vi "Dresden R2R Sputter 03.02.2018 IY24.vi"() -> ()   [LabVIEW 2009] (continued)
                                frame #1 {
                                n17950 = local read "Semi"() -> (w26326:bool)
                                n17951 = case shown="False" w26326 {
                                frame #0 {
                                n17952 = local write "Ch2_PA19"(TRUE ("PA3")) -> ()
                                n17953 = Wait Until Next ms Multiple(millisecond multiple=u32 1000) -> ()  [unwired: 1 out]
                                }
                                frame #1 {
                                }
                                }
                                }
                                }
                              }
                              frame #1 {
                              }
                            }
                          }
                          frame #14 {
                            # "CLOSE CH1-VBV"
                            n17954 = local read "Semi"() -> (w26329:bool)
                            n17955 = case shown="False" w26329 {
                              frame #0 {
                                n17956 = stacked-sequence {
                                frame #0 {
                                n17957 = local read "Semi"() -> (w26330:bool)
                                n17958 = case shown="False" w26330 {
                                frame #0 {
                                n17959 = while {
                                i -> [w26337]
                                stop <- w26331 stop-if-true
                                n17960 = Greater?(x=w26337, y=50) -> (0:w26335:bool)
                                n17961 = case shown="True" w26335 {
                                frame #0 {
                                }
                                frame #1 {
                                n17962 = local write "Semi"(TRUE ("Semi")) -> ()
                                n17963 = local write "Error Message"("Start up process  cancelled\nbecause  CH2-VBV not closed.\nPlease check  CH2-VBV connections." ("Error Message")) -> ()
                                }
                                }
                                n17964 = local read "Ch2_Ch_vbv_di"() -> (w26334:bool)
                                n17965 = case shown="True" w26334 {
                                tunnel: [TRUE FALSE] -> w26333
                                frame #0 {
                                }
                                frame #1 {
                                n17966 = Wait Until Next ms Multiple(millisecond multiple=u32 200) -> ()  [unwired: 1 out]
                                n17967 = local write "Ch2_Ch_vbv_do"(FALSE ("Ch1_Tp_bv_do")) -> ()
                                }
                                }
                                n17968 = local read "Semi"() -> (w26332:bool)
                                n17969 = Or(x=w26333, y=w26332) -> (x .or. y?=w26331:bool)
                                }
                                }
                                frame #1 {
                                }
                                }
                                }
                                frame #1 {
                                n17970 = local read "Semi"() -> (w26344:bool)
                                n17971 = case shown="False" w26344 {
                                frame #0 {
                                n17972 = local write "Ch2_PA20"(TRUE ("PA3")) -> ()
                                n17973 = Wait Until Next ms Multiple(millisecond multiple=u32 1000) -> ()  [unwired: 1 out]
                                }
                                frame #1 {
                                }
                                }
                                }
                                }
                              }
                              frame #1 {
                              }
                            }
                          }
                          frame #15 {
                            # "Close PL-VBV"
                            n17974 = local read "Semi"() -> (w26347:bool)
                            n17975 = case shown="False" w26347 {
                              frame #0 {
                                n17976 = stacked-sequence {
                                frame #0 {
                                n17977 = local read "Semi"() -> (w26348:bool)
                                n17978 = case shown="False" w26348 {
                                frame #0 {
                                n17979 = while {
                                i -> [w26355]
                                stop <- w26349 stop-if-true
                                n17980 = Greater?(x=w26355, y=50) -> (0:w26353:bool)
                                n17981 = case shown="True" w26353 {
                                frame #0 {
                                }
                                frame #1 {
                                n17982 = local write "Semi"(TRUE ("Semi")) -> ()
                                n17983 = local write "Error Message"("Start up process  cancelled\nbecause  PL-VBV not closed.\nPlease check PL2-VBV connections." ("Error Message")) -> ()
                                }
                                }
                                n17984 = local read "Ch2_Pl_vbv_di"() -> (w26352:bool)
                                n17985 = case shown="True" w26352 {
                                tunnel: [TRUE FALSE] -> w26351
                                frame #0 {
                                }
                                frame #1 {
                                n17986 = Wait Until Next ms Multiple(millisecond multiple=u32 200) -> ()  [unwired: 1 out]
                                n17987 = local write "Ch2_Pl_vbv_do"(FALSE ("Ch1_Tp_bv_do")) -> ()
                                }
                                }
                                n17988 = local read "Semi"() -> (w26350:bool)
                                n17989 = Or(x=w26351, y=w26350) -> (x .or. y?=w26349:bool)
                                }
                                }
                                frame #1 {
                                }
                                }
                                }
                                frame #1 {
                                n17990 = local read "Semi"() -> (w26362:bool)
                                n17991 = case shown="False" w26362 {
                                frame #0 {
                                n17992 = local write "Ch2_PA21"(TRUE ("PA3")) -> ()
                                n17993 = Wait Until Next ms Multiple(millisecond multiple=u32 1000) -> ()  [unwired: 1 out]
                                }
                                frame #1 {
                                }
                                }
                                }
                                }
                              }
                              frame #1 {
                              }
                            }
                          }
                          frame #16 {
                            # "OPEN TP-BV"
                            n17994 = local read "Semi"() -> (w26365:bool)
                            n17995 = case shown="False" w26365 {
                              frame #0 {
                                n17996 = stacked-sequence {
                                frame #0 {
                                n17997 = local read "Semi"() -> (w26366:bool)
                                n17998 = case shown="False" w26366 {
                                frame #0 {
                                n17999 = while {
                                i -> [w26373]
                                stop <- w26368 stop-if-true
                                n18000 = Greater?(x=w26373, y=50) -> (0:w26371:bool)
                                n18001 = case shown="True" w26371 {
                                frame #0 {
                                }
                                frame #1 {
                                n18002 = local write "Semi"(TRUE ("Semi")) -> ()
                                n18003 = local write "Error Message"("Start up process  cancelled\nbecause  TP-BV not opened.\nPlease check TP-BV2 connections." ("Error Message")) -> ()
                                }
                                }
                                n18004 = local read "Ch2_Tp_bv_di"() -> (w26367:bool)
                                n18005 = case shown="False" w26367 {
                                tunnel: [FALSE TRUE] -> w26370
                                frame #0 {
                                n18006 = Wait Until Next ms Multiple(millisecond multiple=u32 200) -> ()  [unwired: 1 out]
                                n18007 = local write "Ch2_Tp_bv_do"(TRUE ("Ch1_Tp_bv_do")) -> ()
                                }
                                frame #1 {
                                }
                                }
                                n18008 = local read "Semi"() -> (w26369:bool)
                                n18009 = Or(x=w26370, y=w26369) -> (x .or. y?=w26368:bool)
                                }
                                }
                                frame #1 {
                                }
                                }
                                }
                                frame #1 {
                                n18010 = local read "Semi"() -> (w26380:bool)
                                n18011 = case shown="False" w26380 {
                                frame #0 {
                                n18012 = local write "Ch2_PA22"(TRUE ("PA3")) -> ()
                                n18013 = Wait Until Next ms Multiple(millisecond multiple=u32 1000) -> ()  [unwired: 1 out]
                                }
                                frame #1 {
                                }
                                }
                                }
                                }
                              }
                              frame #1 {
                              }
                            }
                          }
                          frame #17 {
                            # "CLOSE CH-ATM"
                            n18014 = local read "Semi"() -> (w26383:bool)
                            n18015 = case shown="False" w26383 {
                              frame #0 {
                                n18016 = stacked-sequence {
                                frame #0 {
                                n18017 = local read "Semi"() -> (w26384:bool)
                                n18018 = case shown="False" w26384 {
                                frame #0 {
                                n18019 = while {
                                i -> [w26391]
                                stop <- w26385 stop-if-true
                                n18020 = Greater?(x=w26391, y=50) -> (0:w26389:bool)
                                n18021 = case shown="True" w26389 {
                                frame #0 {
                                }
                                frame #1 {
                                n18022 = local write "Semi"(TRUE ("Semi")) -> ()
                                n18023 = local write "Error Message"("Start up process  cancelled\nbecause CH-ATM not closed.\nPlease check CH2-ATM connections." ("Error Message")) -> ()
                                }
                                }
                                n18024 = local read "Ch2_Ch_atm_di"() -> (w26388:bool)
                                n18025 = case shown="True" w26388 {
                                tunnel: [TRUE FALSE] -> w26387
                                frame #0 {
                                }
                                frame #1 {
                                n18026 = Wait Until Next ms Multiple(millisecond multiple=u32 200) -> ()  [unwired: 1 out]
                                n18027 = local write "Ch2_Ch_atm_do"(TRUE ("Ch1_Tp_bv_do")) -> ()
                                }
                                }
                                n18028 = local read "Semi"() -> (w26386:bool)
                                n18029 = Or(x=w26387, y=w26386) -> (x .or. y?=w26385:bool)
                                }
                                }
                                frame #1 {
                                }
                                }
                                }
                                frame #1 {
                                n18030 = local read "Semi"() -> (w26398:bool)
                                n18031 = case shown="False" w26398 {
                                frame #0 {
                                n18032 = local write "Ch2_PA23"(TRUE ("PA3")) -> ()
                                n18033 = Wait Until Next ms Multiple(millisecond multiple=u32 1000) -> ()  [unwired: 1 out]
                                }
                                frame #1 {
                                }
                                }
                                }
                                }
                              }
                              frame #1 {
                              }
                            }
                          }
                          frame #18 {
                            # "CLOSE PL-ATM"
                            n18034 = local read "Semi"() -> (w26401:bool)
                            n18035 = case shown="False" w26401 {
                              frame #0 {
                                n18036 = stacked-sequence {
                                frame #0 {
                                n18037 = local read "Semi"() -> (w26402:bool)
                                n18038 = case shown="False" w26402 {
                                frame #0 {
                                n18039 = while {
                                i -> [w26409]
                                stop <- w26403 stop-if-true
                                n18040 = Greater?(x=w26409, y=50) -> (0:w26407:bool)
                                n18041 = case shown="True" w26407 {
                                frame #0 {
                                }
                                frame #1 {
                                n18042 = local write "Semi"(TRUE ("Semi")) -> ()
                                n18043 = local write "Error Message"("Start up process  cancelled\nbecause  PL-ATM not closed.\nPlease check PL-ATM2 connections." ("Error Message")) -> ()
                                }
                                }
                                n18044 = local read "Ch2_Pl_atm_di"() -> (w26406:bool)
                                n18045 = case shown="True" w26406 {
                                tunnel: [TRUE FALSE] -> w26405
                                frame #0 {
                                }
                                frame #1 {
                                n18046 = Wait Until Next ms Multiple(millisecond multiple=u32 200) -> ()  [unwired: 1 out]
                                n18047 = local write "Ch2_Pl_atm_do"(TRUE ("Ch1_Tp_bv_do")) -> ()
                                }
                                }
                                n18048 = local read "Semi"() -> (w26404:bool)
                                n18049 = Or(x=w26405, y=w26404) -> (x .or. y?=w26403:bool)
                                }
                                }
                                frame #1 {
                                }
                                }
                                }
                                frame #1 {
                                n18050 = local read "Semi"() -> (w26416:bool)
                                n18051 = case shown="False" w26416 {
                                frame #0 {
                                n18052 = local write "Ch2_PA24"(TRUE ("PA3")) -> ()
                                n18053 = Wait Until Next ms Multiple(millisecond multiple=u32 1000) -> ()  [unwired: 1 out]
                                }
                                frame #1 {
                                }
                                }
                                }
                                }
                              }
                              frame #1 {
                              }
                            }
                          }
                          frame #19 {
                            # "START MP"
                            n18054 = local read "Semi"() -> (w26419:bool)
                            n18055 = case shown="False" w26419 {
                              frame #0 {
                                n18056 = stacked-sequence {
                                frame #0 {
                                n18057 = local read "Semi"() -> (w26420:bool)
                                n18058 = case shown="False" w26420 {
                                frame #0 {
                                n18059 = while {
                                i -> [w26427]
                                stop <- w26421 stop-if-true
                                n18060 = Greater?(x=w26427, y=50) -> (0:w26425:bool)
                                n18061 = case shown="True" w26425 {
                                frame #0 {
                                }
                                frame #1 {
                                n18062 = local write "Semi"(TRUE ("Semi")) -> ()
                                n18063 = local write "Error Message"("Start up process  cancelled\nbecause MP not started.\nPlease check MP2 connections." ("Error Message")) -> ()
                                }
                                }
                                n18064 = local read "Ch2_Mp_di"() -> (w26424:bool)
                                n18065 = case shown="False" w26424 {
                                tunnel: [FALSE TRUE] -> w26423
                                frame #0 {
                                n18066 = Wait Until Next ms Multiple(millisecond multiple=u32 200) -> ()  [unwired: 1 out]
                                n18067 = local write "Ch2_Mp_do"(TRUE ("Ch1_Tp_bv_do")) -> ()
                                }
                                frame #1 {
                                }
                                }
                                n18068 = local read "Semi"() -> (w26422:bool)
                                n18069 = Or(x=w26423, y=w26422) -> (x .or. y?=w26421:bool)
                                }
                                }
                                frame #1 {
                                }
                                }
                                }
                                frame #1 {
                                n18070 = local read "Semi"() -> (w26434:bool)
                                n18071 = case shown="False" w26434 {
                                frame #0 {
                                n18072 = local write "Ch2_PA25"(TRUE ("PA3")) -> ()
                                n18073 = Wait Until Next ms Multiple(millisecond multiple=u32 1000) -> ()  [unwired: 1 out]
                                }
                                frame #1 {
                                }
                                }
                                }
                                }
                              }
                              frame #1 {
                              }
                            }
                          }
                          frame #20 {
                            # "START TP"
                            n18074 = local read "Semi"() -> (w26437:bool)
                            n18075 = case shown="False" w26437 {
                              frame #0 {
                                n18076 = stacked-sequence {
                                frame #0 {
                                n18077 = local read "Semi"() -> (w26438:bool)
                                n18078 = case shown="False" w26438 {
                                frame #0 {
                                n18079 = stacked-sequence {
                                frame #0 {
                                n18080 = local read "Semi"() -> (w26439:bool)
                                n18081 = case shown="False" w26439 {
                                frame #0 {
                                n18082 = local write "Tp2_auto_start"(TRUE ("Tp1_auto_start")) -> ()
                                }
                                frame #1 {
                                }
                                }
                                }
                                frame #1 {
                                n18083 = local read "Semi"() -> (w26441:bool)
                                n18084 = case shown="False" w26441 {
                                frame #0 {
                                n18085 = Wait (ms)(milliseconds to wait=u32 1000) -> ()  [unwired: 1 out]
                                }
                                frame #1 {
                                }
                                }
                                }
                                frame #2 {
                                n18086 = local read "Semi"() -> (w26443:bool)
                                n18087 = case shown="False" w26443 {
                                frame #0 {
                                n18088 = local write "Tp2_auto_start"(TRUE ("Tp1_auto_start")) -> ()
                                }
                                frame #1 {
                                }
                                }
                                }
                                }
                                }
                                frame #1 {
                                }
                                }
                                }
                                frame #1 {
                                n18089 = local read "Semi"() -> (w26445:bool)
                                n18090 = case shown="False" w26445 {
                                frame #0 {
                                n18091 = local write "Ch2_PA30"(TRUE ("PA3")) -> ()
                                n18092 = Wait Until Next ms Multiple(millisecond multiple=u32 1000) -> ()  [unwired: 1 out]
                                }
                                frame #1 {
                                }
                                }
                                }
                                }
                              }
                              frame #1 {
                              }
                            }
                          }
                          frame #21 {
                            # "CHECK PL-PRESSURE"
                            n18093 = local read "Semi"() -> (w26448:bool)
                            n18094 = case shown="False" w26448 {
                              frame #0 {
                                n18095 = stacked-sequence {
                                frame #0 {
                                n18096 = local read "Semi"() -> (w26449:bool)
                                n18097 = case shown="False" w26449 {
                                frame #0 {
                                n18098 = while {
                                i -> [w26458]
                                stop <- w26453 stop-if-true
                                n18099 = Greater?(x=w26458, y=1200) -> (0:w26456:bool)
                                n18100 = case shown="True" w26456 {
                                frame #0 {
                                }
                                frame #1 {
                                n18101 = local write "Semi"(TRUE ("Semi")) -> ()
                                n18102 = local write "Error Message"("Start up process was cancelled.\nPlease check Pipeline \nvacuum connections." ("Error Message")) -> ()
                                }
                                }
                                n18103 = local read "Pl_pg_press_ch2"() -> (w26452:dbl)
                                n18104 = Less?(x=w26452, y=0.9) -> (x < y?=w26450:bool)
                                n18105 = case shown="False" w26450 {
                                tunnel: [FALSE TRUE] -> w26455
                                frame #0 {
                                n18106 = Wait Until Next ms Multiple(millisecond multiple=u32 500) -> ()  [unwired: 1 out]
                                }
                                frame #1 {
                                }
                                }
                                n18107 = local read "Semi"() -> (w26454:bool)
                                n18108 = Or(x=w26455, y=w26454) -> (x .or. y?=w26453:bool)
                                }
                                }
                                frame #1 {
                                }
                                }
                                }
                                frame #1 {
                                n18109 = local read "Semi"() -> (w26464:bool)
                                n18110 = case shown="False" w26464 {
                                frame #0 {
                                n18111 = local write "Ch2_PA26"(TRUE ("PA3")) -> ()
                                n18112 = Wait Until Next ms Multiple(millisecond multiple=u32 1000) -> ()  [unwired: 1 out]
                                }
                                frame #1 {
                                }
                                }
                                }
                                }
                              }
                              frame #1 {
                              }
                            }
                          }
                          frame #22 {
                            # "CHECK CH-PRESSURE"
                            n18113 = local read "Semi"() -> (w26467:bool)
                            n18114 = case shown="False" w26467 {
                              frame #0 {
                                n18115 = stacked-sequence {
                                frame #0 {
                                n18116 = local read "Semi"() -> (w26468:bool)
                                n18117 = case shown="False" w26468 {
                                frame #0 {
                                n18118 = while {
                                i -> [w26477]
                                stop <- w26472 stop-if-true
                                n18119 = Greater?(x=w26477, y=1200) -> (0:w26475:bool)
                                n18120 = case shown="True" w26475 {
                                frame #0 {
                                }
                                frame #1 {
                                n18121 = local write "Semi"(TRUE ("Semi")) -> ()
                                n18122 = local write "Error Message"("Start up process was cancelled.\nPlease check chamber \nvacuum connections." ("Error Message")) -> ()
                                }
                                }
                                n18123 = local read "Ch2_pressure"() -> (w26471:dbl)
                                n18124 = Less?(x=w26471, y=0.9) -> (x < y?=w26469:bool)
                                n18125 = case shown="False" w26469 {
                                tunnel: [FALSE TRUE] -> w26474
                                frame #0 {
                                n18126 = Wait Until Next ms Multiple(millisecond multiple=u32 500) -> ()  [unwired: 1 out]
                                }
                                frame #1 {
                                }
                                }
                                n18127 = local read "Semi"() -> (w26473:bool)
                                n18128 = Or(x=w26474, y=w26473) -> (x .or. y?=w26472:bool)
                                }
                                }
                                frame #1 {
                                }
                                }
                                }
                                frame #1 {
                                n18129 = local read "Semi"() -> (w26483:bool)
                                n18130 = case shown="False" w26483 {
                                frame #0 {
                                n18131 = local write "Ch2_PA27"(TRUE ("PA3")) -> ()
                                n18132 = Wait Until Next ms Multiple(millisecond multiple=u32 1000) -> ()  [unwired: 1 out]
                                }
                                frame #1 {
                                }
                                }
                                }
                                }
                              }
                              frame #1 {
                              }
                            }
                          }
                          frame #23 {
                            # "OPEN BG-BV"
                            n18133 = local read "Semi"() -> (w26486:bool)
                            n18134 = case shown="False" w26486 {
                              frame #0 {
                                n18135 = stacked-sequence {
                                frame #0 {
                                n18136 = local read "Semi"() -> (w26487:bool)
                                n18137 = case shown="False" w26487 {
                                frame #0 {
                                n18138 = while {
                                i -> [w26494]
                                stop <- w26489 stop-if-true
                                n18139 = Greater?(x=w26494, y=50) -> (0:w26492:bool)
                                n18140 = case shown="True" w26492 {
                                frame #0 {
                                }
                                frame #1 {
                                n18141 = local write "Semi"(TRUE ("Semi")) -> ()
                                n18142 = local write "Error Message"("Start up process  cancelled\nbecause  BG-BV not opened.\nPlease check BG-BV2 connections." ("Error Message")) -> ()
                                }
                                }
                                n18143 = local read "Ch2_Bg_bv_di"() -> (w26488:bool)
                                n18144 = case shown="False" w26488 {
                                tunnel: [FALSE TRUE] -> w26491
                                frame #0 {
                                n18145 = Wait Until Next ms Multiple(millisecond multiple=u32 200) -> ()  [unwired: 1 out]
                                n18146 = local write "Ch2_Bg_bv_do"(TRUE ("Ch1_Tp_bv_do")) -> ()
                                }
                                frame #1 {
                                }
                                }
                                n18147 = local read "Semi"() -> (w26490:bool)
                                n18148 = Or(x=w26491, y=w26490) -> (x .or. y?=w26489:bool)
                                }
                                }
                                frame #1 {
                                }
                                }
                                }
                                frame #1 {
                                n18149 = local read "Semi"() -> (w26501:bool)
                                n18150 = case shown="False" w26501 {
                                frame #0 {
                                n18151 = local write "Ch2_PA28"(TRUE ("PA3")) -> ()
                                n18152 = Wait Until Next ms Multiple(millisecond multiple=u32 1000) -> ()  [unwired: 1 out]
                                }
                                frame #1 {
                                }
                                }
                                }
                                }
                              }
                              frame #1 {
                              }
                            }
                          }
                          frame #24 {
                            # "CHECK CH-PRESSURE"
                            n18153 = local read "Semi"() -> (w26504:bool)
                            n18154 = case shown="False" w26504 {
                              frame #0 {
                                n18155 = stacked-sequence {
                                frame #0 {
                                n18156 = local read "Semi"() -> (w26505:bool)
                                n18157 = case shown="False" w26505 {
                                frame #0 {
                                n18158 = while {
                                i -> [w26514]
                                stop <- w26509 stop-if-true
                                n18159 = Greater?(x=w26514, y=600) -> (0:w26512:bool)
                                n18160 = case shown="True" w26512 {
                                frame #0 {
                                }
                                frame #1 {
                                n18161 = local write "Semi"(TRUE ("Semi")) -> ()
                                n18162 = local write "Error Message"("Start up process was cancelled.\nPlease check chamber \nvacuum connections." ("Error Message")) -> ()
                                }
                                }
                                n18163 = local read "Ch2_pressure"() -> (w26508:dbl)
                                n18164 = Less?(x=w26508, y=0.9) -> (x < y?=w26506:bool)
                                n18165 = case shown="False" w26506 {
                                tunnel: [FALSE TRUE] -> w26511
                                frame #0 {
                                n18166 = Wait Until Next ms Multiple(millisecond multiple=u32 500) -> ()  [unwired: 1 out]
                                }
                                frame #1 {
                                }
                                }
                                n18167 = local read "Semi"() -> (w26510:bool)
                                n18168 = Or(x=w26511, y=w26510) -> (x .or. y?=w26509:bool)
                                }
                                }
                                frame #1 {
                                }
                                }
                                }
                                frame #1 {
                                n18169 = local read "Semi"() -> (w26520:bool)
                                n18170 = case shown="False" w26520 {
                                frame #0 {
                                n18171 = local write "Ch2_PA29"(TRUE ("PA3")) -> ()
                                n18172 = Wait Until Next ms Multiple(millisecond multiple=u32 1000) -> ()  [unwired: 1 out]
                                }
                                frame #1 {
                                }
                                }
                                }
                                }
                              }
                              frame #1 {
                              }
                            }
                          }
                          frame #25 {
                            # "START TP"
                            n18173 = local read "Semi"() -> (w26523:bool)
                            n18174 = case shown="False" w26523 {
                              frame #0 {
                                n18175 = stacked-sequence {
                                frame #0 {
                                n18176 = local read "Semi"() -> (w26524:bool)
                                n18177 = case shown="False" w26524 {
                                frame #0 {
                                n18178 = stacked-sequence {
                                frame #0 {
                                n18179 = local read "Semi"() -> (w26525:bool)
                                n18180 = case shown="False" w26525 {
                                frame #0 {
                                n18181 = local write "Tp2_auto_start"(TRUE ("Tp1_auto_start")) -> ()
                                }
                                frame #1 {
                                }
                                }
                                }
                                frame #1 {
                                n18182 = local read "Semi"() -> (w26527:bool)
                                n18183 = case shown="False" w26527 {
                                frame #0 {
                                n18184 = Wait (ms)(milliseconds to wait=u32 1000) -> ()  [unwired: 1 out]
                                }
                                frame #1 {
                                }
                                }
                                }
                                frame #2 {
                                n18185 = local read "Semi"() -> (w26529:bool)
                                n18186 = case shown="False" w26529 {
                                frame #0 {
                                n18187 = while {
                                i -> [w26535]
                                stop <- w26531 stop-if-true
                                n18188 = local read "TP2_working"() -> (w26533:bool)
                                n18189 = Greater?(x=w26535, y=120) -> (0:w26534:bool)
                                n18190 = local read "Semi"() -> (w26532:bool)
                                n18191 = Compound Arithmetic op=OR(w26532, w26533, w26534) -> (w26531:bool)
                                n18192 = Wait (ms)(milliseconds to wait=u32 500) -> ()  [unwired: 1 out]
                                }
                                }
                                frame #1 {
                                }
                                }
                                }
                                frame #3 {
                                n18193 = local read "Semi"() -> (w26537:bool)
                                n18194 = case shown="False" w26537 {
                                frame #0 {
                                n18195 = local read "TP2_working"() -> (w26538:bool)
                                n18196 = case shown="False" w26538 {
                                frame #0 {
                                n18197 = local write "Tp2_auto_start"(TRUE ("Pc_bv1_auto_open")) -> ()
                                }
                                frame #1 {
                                }
                                }
                                }
                                frame #1 {
                                }
                                }
                                }
                                frame #4 {
                                n18198 = local read "Semi"() -> (w26540:bool)
                                n18199 = case shown="False" w26540 {
                                frame #0 {
                                n18200 = local read "TP2_working"() -> (w26541:bool)
                                n18201 = case shown="False" w26541 {
                                frame #0 {
                                n18202 = Wait (ms)(milliseconds to wait=u32 1000) -> ()  [unwired: 1 out]
                                }
                                frame #1 {
                                }
                                }
                                }
                                frame #1 {
                                }
                                }
                                }
                                frame #5 {
                                n18203 = local read "Semi"() -> (w26543:bool)
                                n18204 = case shown="False" w26543 {
                                frame #0 {
                                n18205 = while {
                                i -> [w26549]
                                stop <- w26545 stop-if-true
                                n18206 = local read "TP2_working"() -> (w26547:bool)
                                n18207 = Greater?(x=w26549, y=120) -> (0:w26548:bool)
                                n18208 = local read "Semi"() -> (w26546:bool)
                                n18209 = Compound Arithmetic op=OR(w26546, w26547, w26548) -> (w26545:bool)
                                n18210 = Wait (ms)(milliseconds to wait=u32 500) -> ()  [unwired: 1 out]
                                }
                                }
                                frame #1 {
                                }
                                }
                                }
                                frame #6 {
                                n18211 = local read "Semi"() -> (w26551:bool)
                                n18212 = case shown="False" w26551 {
                                frame #0 {
                                n18213 = local read "TP2_working"() -> (w26552:bool)
                                n18214 = case shown="False" w26552 {
                                frame #0 {
                                n18215 = local write "Error Message"("Start up process  cancelled\nbecause  TP not started.\nPlease check TP2 connections." ("Error Message")) -> ()
                                n18216 = Wait (ms)(milliseconds to wait=u32 1000) -> ()  [unwired: 1 out]
                                }
                                frame #1 {
                                }
                                }
                                }
                                frame #1 {
                                }
                                }
                                }
                                }
                                }
                                frame #1 {
                                }
                                }
                                }
                                frame #1 {
                                n18217 = local read "Semi"() -> (w26555:bool)
                                n18218 = case shown="False" w26555 {
                                frame #0 {
                                n18219 = local write "Ch2_PA30"(TRUE ("PA3")) -> ()
                                n18220 = Wait Until Next ms Multiple(millisecond multiple=u32 1000) -> ()  [unwired: 1 out]
                                }
                                frame #1 {
                                }
                                }
                                }
                                }
                              }
                              frame #1 {
                              }
                            }
                          }
                          frame #26 {
                            # "CHECK CH-PRESSURE"
                            n18221 = local read "Semi"() -> (w26558:bool)
                            n18222 = case shown="False" w26558 {
                              frame #0 {
                                n18223 = stacked-sequence {
                                frame #0 {
                                n18224 = local read "Semi"() -> (w26559:bool)
                                n18225 = case shown="False" w26559 {
                                frame #0 {
                                n18226 = while {
                                i -> [w26568]
                                stop <- w26563 stop-if-true
                                n18227 = Greater?(x=w26568, y=240) -> (0:w26566:bool)
                                n18228 = case shown="True" w26566 {
                                frame #0 {
                                }
                                frame #1 {
                                n18229 = local write "Semi"(TRUE ("Semi")) -> ()
                                n18230 = local write "Error Message"("Start up process was cancelled.\nPlease check chamber \nvacuum connections." ("Error Message")) -> ()
                                }
                                }
                                n18231 = local read "Ch2_pressure"() -> (w26562:dbl)
                                n18232 = Less?(x=w26562, y=0.9) -> (x < y?=w26560:bool)
                                n18233 = case shown="False" w26560 {
                                tunnel: [FALSE TRUE] -> w26565
                                frame #0 {
                                n18234 = Wait Until Next ms Multiple(millisecond multiple=u32 500) -> ()  [unwired: 1 out]
                                }
                                frame #1 {
                                }
                                }
                                n18235 = local read "Semi"() -> (w26564:bool)
                                n18236 = Or(x=w26565, y=w26564) -> (x .or. y?=w26563:bool)
                                }